vi "rs3_cull_obj2.vi"(7 "file path (dialog if empty)":path=path "C:/ProgramData/Obj_and_PNG_Recording/FacePointCloud_4.obj", 10 "all faces input":i32[][](array[numeric])=array65200x3[195600 elements], 11 "vertices":dbl[][](array[numeric])=array32964x6[197784 elements]) -> (2 "New Faces (proper index)":dbl[][](array[numeric]), 3 "new vertices":dbl[][](array[numeric]))   [LabVIEW 2017, in "libRealSense3.lvlib"]
uses:
  <vilib>/Utility/file.llb/Write Delimited Spreadsheet (string).vi
  libRealSense3.lvlib
panel:
  out "depth array":dbl[](array[numeric])
  out "Good faces":bool[](array[boolean])
  out "Valid vertices":bool[](array[boolean])
  out "New valid faces":i32[][](array[numeric])
  out "Offset":dbl[](array[numeric])
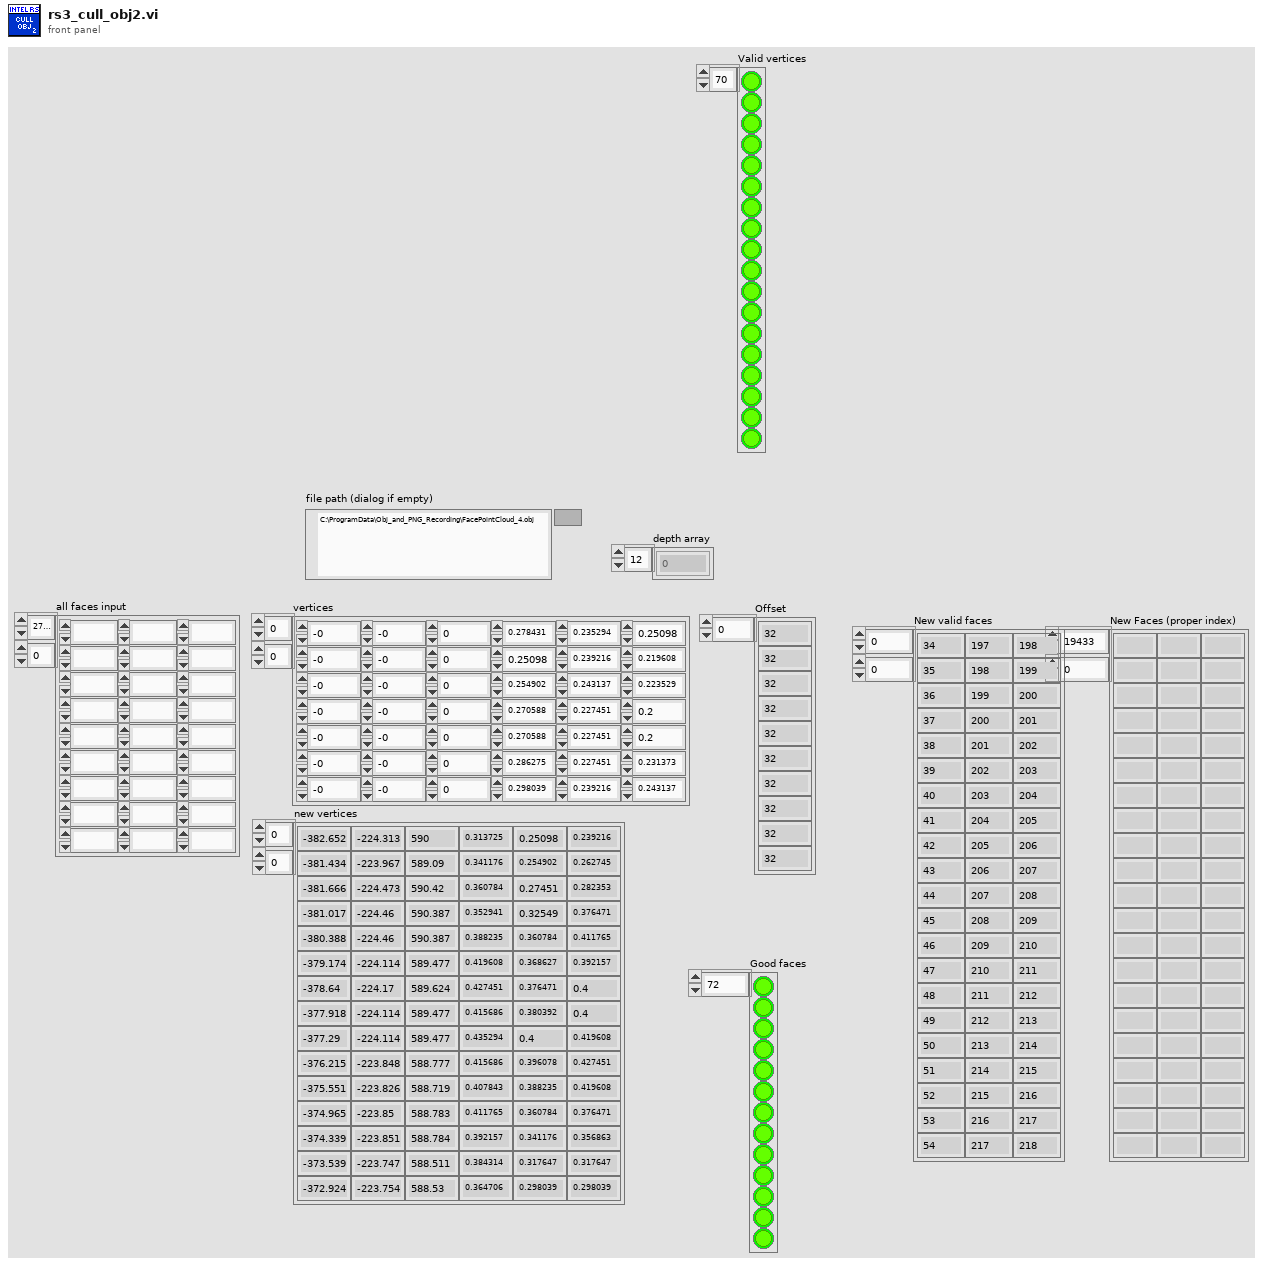
[diagram p1: front panel]
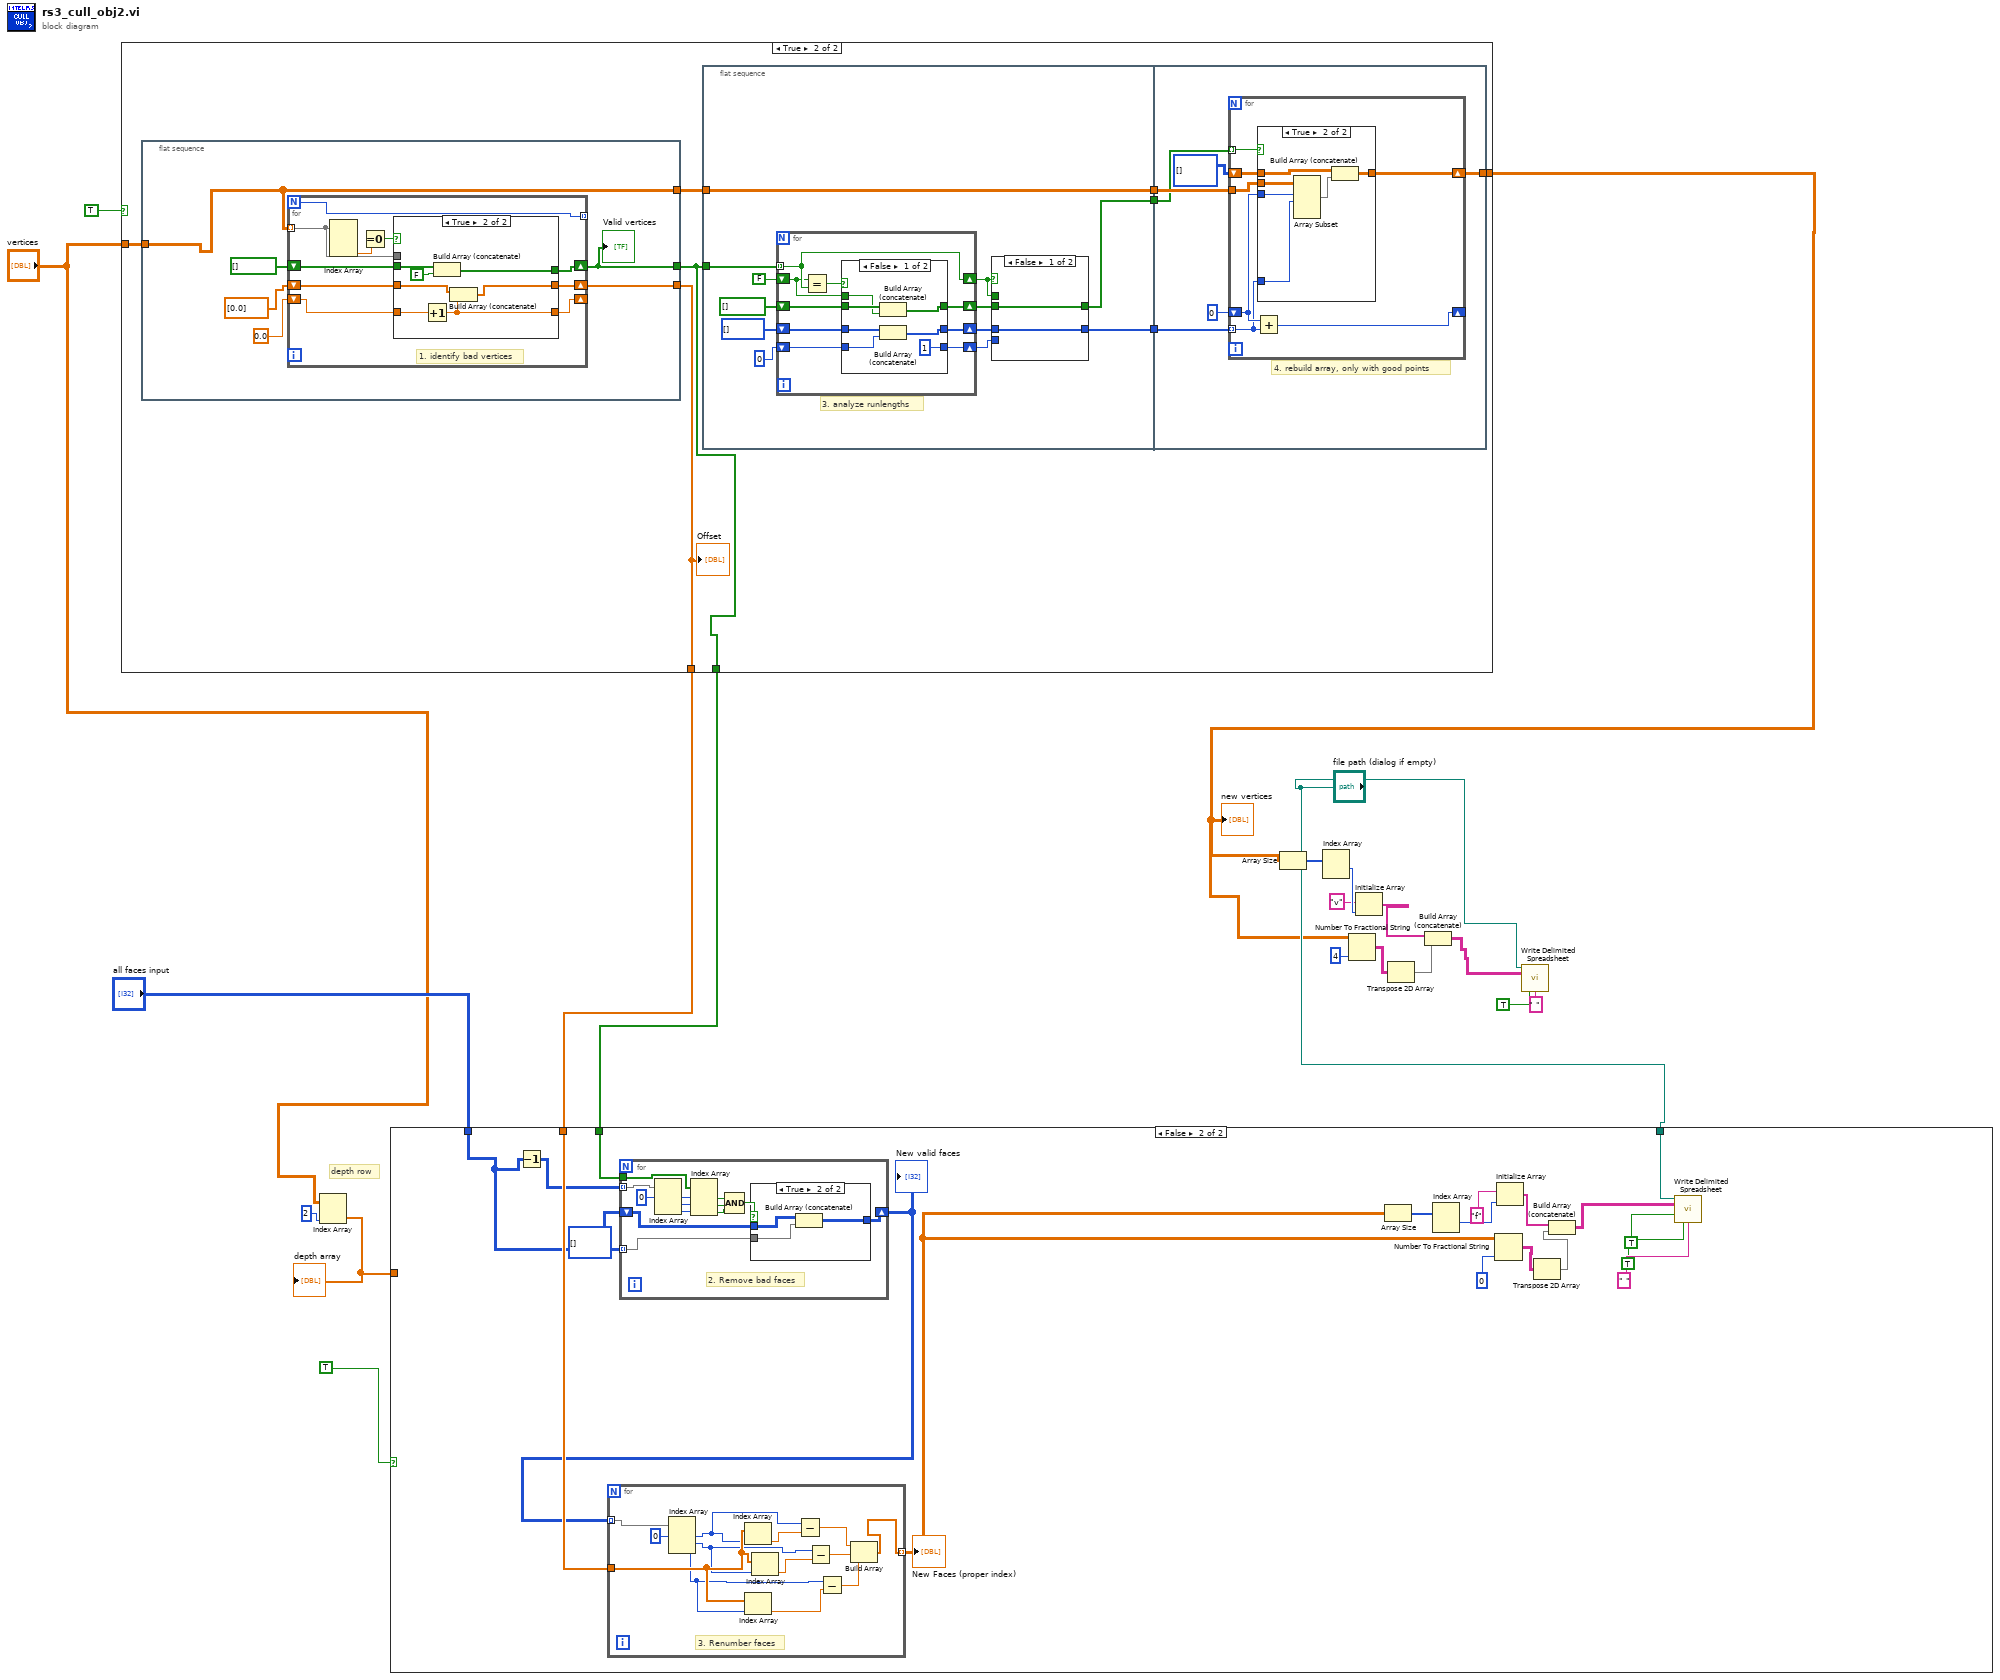
[diagram p0: block diagram]
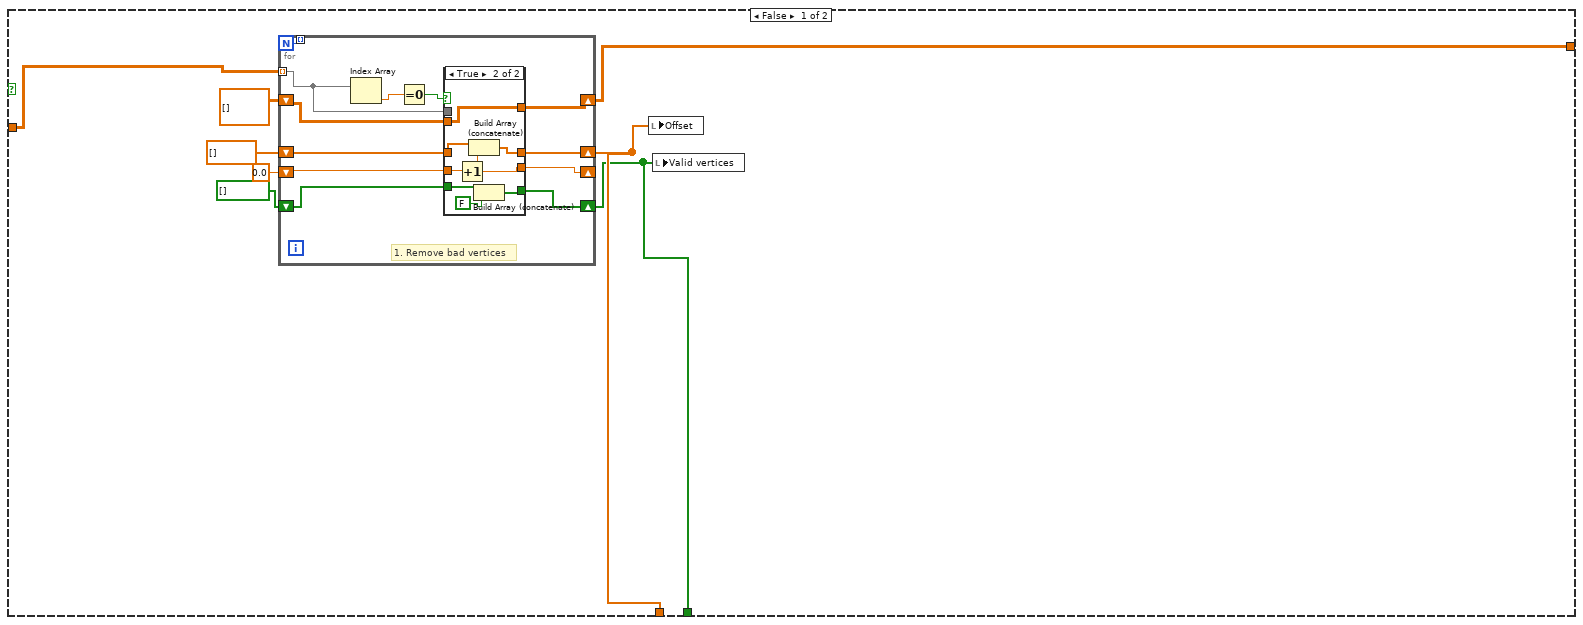
[diagram p2: hidden frame]
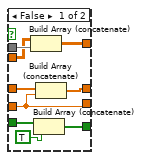
[diagram p3: hidden frame]
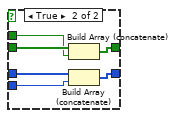
[diagram p4: hidden frame]
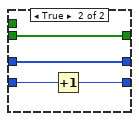
[diagram p5: hidden frame]
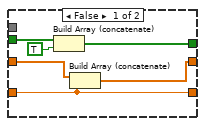
[diagram p7: hidden frame]
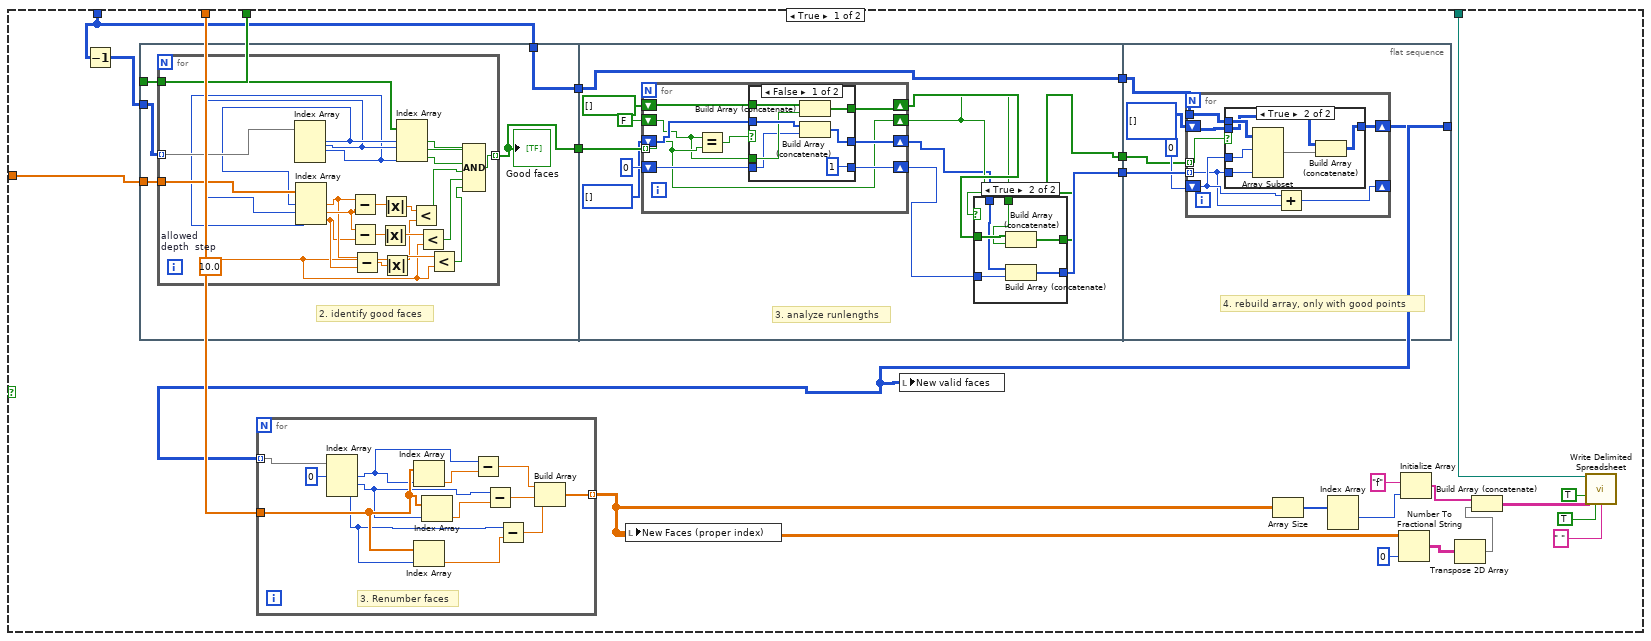
[diagram p8: hidden frame]
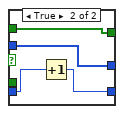
[diagram p10: hidden frame]
diagram:
  # "depth row"
  n1 = case shown="True" TRUE {
    tunnel: [w22 w61] -> w7
    tunnel: "vertices" -> [w24 w60]
    tunnel: [w23 w58] -> w5
    tunnel: [w21 w59] -> w4
    frame False {
      n2 = for {
        N -> [w31]
        tunnel: w24 -> [w40] mode=indexing
        shift-right: [w39] -> w22
        shift-left: dbl[][] [] -> [w37]
        shift-right: [w32] -> w23
        shift-left: dbl[] [] -> [w35]
        shift-right: [w33] -> _
        shift-left: 0.0 -> [w34]
        tunnel: [w31] -> _ mode=indexing
        shift-right: [w29] -> w21
        shift-left: bool[] [] -> [w30]
        # "1. Remove bad vertices"
        n3 = Index Array(array=w40) -> (element=w36:dbl)  [unwired: 1 in]
        n4 = Equal To 0?(x=w36) -> (x = 0?=w38:bool)
        n5 = case shown="True" w38 {
          tunnel: w40 -> [w49 _]
          tunnel: [w48 w57] -> w39
          tunnel: w37 -> [w47 w57]
          tunnel: w35 -> [w46 w52]
          tunnel: w34 -> [w45 w56]
          tunnel: [w45 w51] -> w33
          tunnel: [w44 w50] -> w32
          tunnel: [w43 w53] -> w29
          tunnel: w30 -> [w41 w55]
          frame False {
            n6 = Build Array (concatenate)(w47, w49) -> (w48:dbl[][])
            n7 = Build Array (concatenate)(w41, TRUE) -> (w43:bool[])
            n8 = Build Array (concatenate)(w46, w45) -> (w44:dbl[])
          }
          frame True {
            n9 = Increment(x=w56) -> (x+1=w51:dbl)
            n10 = Build Array (concatenate)(w52, w51) -> (w50:dbl[])
            n11 = Build Array (concatenate)(w55, FALSE) -> (w53:bool[])
          }
        }
      }
      n12 = local write "Offset"(w23) -> ()
      n13 = local write "Valid vertices"(w21) -> ()
    }
    frame True {
      n14 = flat-sequence {
        tunnel: [w130] -> w59
        tunnel: [w129] -> w62
        tunnel: w60 -> [w129]
        tunnel: [w126] -> w58
        frame #0 {
          n15 = for {
            N -> [w139]
            tunnel: w129 -> [w141] mode=indexing
            tunnel: [w139] -> _ mode=indexing
            shift-right: [w137] -> w130
            shift-left: bool[] [] -> [w138]
            shift-right: [w133] -> w126
            shift-left: dbl[] [0.0] -> [w135]
            shift-right: [w132] -> _
            shift-left: 0.0 -> [w134]
            # "1. identify bad vertices"
            n16 = Index Array(array=w141) -> (element #3=w136:dbl)  [unwired: 3 in, 2 out]
            n17 = Equal To 0?(x=w136) -> (x = 0?=w140:bool)
            n18 = case shown="True" w140 {
              tunnel: w141 -> [_ _]
              tunnel: [w147 w152] -> w137
              tunnel: w138 -> [w145 w154]
              tunnel: w135 -> [w144 w151]
              tunnel: w134 -> [w142 w149]
              tunnel: [w143 w150] -> w133
              tunnel: [w142 w148] -> w132
              frame False {
                n19 = Build Array (concatenate)(w145, TRUE) -> (w147:bool[])
                n20 = Build Array (concatenate)(w144, w142) -> (w143:dbl[])
              }
              frame True {
                n21 = Increment(x=w149) -> (x+1=w148:dbl)
                n22 = Build Array (concatenate)(w154, FALSE) -> (w152:bool[])
                n23 = Build Array (concatenate)(w151, w148) -> (w150:dbl[])
              }
            }
          }
          "Valid vertices" <- w130
        }
      }
      n24 = flat-sequence {
        tunnel: [w67] -> w65
        tunnel: [w68] -> w64
        tunnel: [w69] -> w63
        tunnel: w62 -> [w67]
        tunnel: w59 -> [w66]
        tunnel: w65 -> [w111]
        tunnel: w64 -> [w108]
        tunnel: w63 -> [w110]
        tunnel: [w106] -> w61
        frame #0 {
          # "3. analyze runlengths"
          n25 = for {
            tunnel: w66 -> [w89] mode=indexing
            shift-right: [w89] -> w72
            shift-left: FALSE -> [w86]
            shift-right: [w93] -> w70
            shift-left: 0 -> [w94]
            shift-right: [w92] -> w71
            shift-left: i32[] [] -> [w91]
            shift-right: [w87] -> w73
            shift-left: bool[] [] -> [w88]
            n26 = Equal?(x=w86, y=w89) -> (x = y?=w90:bool)
            n27 = case shown="False" w90 {
              tunnel: w94 -> [w95 w105]
              tunnel: [1 w104] -> w93
              tunnel: [w100 w103] -> w92
              tunnel: w91 -> [w99 w103]
              tunnel: w88 -> [w98 w102]
              tunnel: [w97 w102] -> w87
              tunnel: w86 -> [w96 _]
              frame False {
                n28 = Build Array (concatenate)(w98, w96) -> (w97:bool[])
                n29 = Build Array (concatenate)(w99, w95) -> (w100:i32[])
              }
              frame True {
                n30 = Increment(x=w105) -> (x+1=w104:i32)
              }
            }
          }
          n31 = case shown="False" w72 {
            tunnel: w73 -> [w79 w85]
            tunnel: w72 -> [_ w84]
            tunnel: w71 -> [w78 w83]
            tunnel: w70 -> [_ w82]
            tunnel: [w78 w81] -> w69
            tunnel: [w79 w80] -> w68
            frame False {
            }
            frame True {
              n32 = Build Array (concatenate)(w85, w84) -> (w80:bool[])
              n33 = Build Array (concatenate)(w83, w82) -> (w81:i32[])
            }
          }
        }
        frame #1 {
          # "4. rebuild array, only with good points"
          n34 = for {
            shift-right: [w116] -> _
            shift-left: 0 -> [w117]
            tunnel: w111 -> [w118]
            tunnel: w110 -> [w115] mode=indexing
            shift-right: [w112] -> w106
            shift-left: i32[][] [] ("all faces input") -> [w114]
            tunnel: w108 -> [w113] mode=indexing
            n35 = Add(x=w117, y=w115) -> (x+y=w116:i32)
            n36 = case shown="True" w113 {
              tunnel: w118 -> [_ w125]
              tunnel: w117 -> [_ w124]
              tunnel: w115 -> [_ w122]
              tunnel: w114 -> [w119 w120]
              tunnel: [w119 w121] -> w112
              frame False {
              }
              frame True {
                n37 = Array Subset(array=w125, index (row)=w124, length (row)=w122) -> (w123:dbl[][])  [unwired: 2 in]
                n38 = Build Array (concatenate)(w120, w123) -> (w121:dbl[][])
              }
            }
          }
        }
      }
      "Offset" <- w58
    }
  }
  "new vertices" <- w7
  n39 = Index Array(array="vertices", index (col)=2 ("index (row)")) -> (element=w2:dbl[])  [unwired: 1 in]
  "depth array" <- w2
  n40 = case shown="False" TRUE {
    tunnel: w4 -> [w160 w297]
    tunnel: "file path (dialog if empty)" -> [w169 w287]
    tunnel: w5 -> [w166 w284]
    tunnel: "all faces input" -> [w158 w281]
    tunnel: w2 -> [w155 _]
    frame True {
      n41 = Decrement(x=w158) -> (x-1=w159:i32[][])
      n42 = flat-sequence {
        tunnel: w160 -> [w183]
        tunnel: w159 -> [w182]
        tunnel: [w181] -> w165
        tunnel: w158 -> [w181]
        tunnel: [w180] -> w164
        tunnel: w155 -> [w179]
        tunnel: w165 -> [w215]
        tunnel: w164 -> [w218]
        tunnel: [w215] -> w163
        tunnel: [w207] -> w162
        tunnel: [w208] -> w161
        tunnel: w163 -> [w252]
        tunnel: w162 -> [w249]
        tunnel: w161 -> [w251]
        tunnel: [w247] -> w157
        frame #0 {
          # "2. identify good faces"
          n43 = for {
            tunnel: w182 -> [w206] mode=indexing
            tunnel: w183 -> [w205]
            tunnel: [w201] -> w180 mode=indexing
            tunnel: w179 -> [w200]
            w192 = 10.0  # allowed  depth  step
            n44 = Index Array(array=w206) -> (element #1=w186:i32, element #2=w184:i32, element #3=w185:i32)  [unwired: 3 in]
            n45 = Index Array(array=w200, index #1=w186, index #2=w185, index #3=w184) -> (element #1=w198:dbl, element #2=w199:dbl, element #3=w197:dbl)
            n46 = Subtract(x=w198, y=w199) -> (x-y=w191:dbl)
            n47 = Subtract(x=w199, y=w197) -> (x-y=w196:dbl)
            n48 = Subtract(x=w198, y=w197) -> (x-y=w195:dbl)
            n49 = Absolute Value(x=w196) -> (abs(x)=w194:dbl)
            n50 = Absolute Value(x=w191) -> (abs(x)=w190:dbl)
            n51 = Absolute Value(x=w195) -> (abs(x)=w193:dbl)
            n52 = Index Array(array=w205, index #1=w186, index #2=w184, index #3=w185) -> (element #1=w204:bool, element #2=w203:bool, element #3=w202:bool)
            n53 = Less?(x=w190, y=w192) -> (x < y?=w189:bool)
            n54 = Less?(x=w194, y=w192) -> (x < y?=w188:bool)
            n55 = Less?(x=w193, y=w192) -> (x < y?=w187:bool)
            n56 = Compound Arithmetic op=AND(w204, w203, w202, w189, w188, w187) -> (w201:bool)
          }
          "Good faces" <- w180
        }
        frame #1 {
          # "3. analyze runlengths"
          n57 = for {
            tunnel: w218 -> [w230] mode=indexing
            shift-right: [w230] -> w211
            shift-left: FALSE -> [w227]
            shift-right: [w234] -> w209
            shift-left: 0 -> [w235]
            shift-right: [w233] -> w210
            shift-left: i32[] [] -> [w232]
            shift-right: [w228] -> w212
            shift-left: bool[] [] -> [w229]
            n58 = Equal?(x=w227, y=w230) -> (x = y?=w231:bool)
            n59 = case shown="False" w231 {
              tunnel: w235 -> [w236 w246]
              tunnel: [1 w245] -> w234
              tunnel: [w241 w244] -> w233
              tunnel: w232 -> [w240 w244]
              tunnel: w229 -> [w239 w243]
              tunnel: [w238 w243] -> w228
              tunnel: w227 -> [w237 _]
              frame False {
                n60 = Build Array (concatenate)(w239, w237) -> (w238:bool[])
                n61 = Build Array (concatenate)(w240, w236) -> (w241:i32[])
              }
              frame True {
                n62 = Increment(x=w246) -> (x+1=w245:i32)
              }
            }
          }
          n63 = case shown="True" w211 {
            tunnel: w212 -> [w220 w226]
            tunnel: w211 -> [_ w225]
            tunnel: w210 -> [w219 w224]
            tunnel: w209 -> [_ w223]
            tunnel: [w219 w222] -> w208
            tunnel: [w220 w221] -> w207
            frame False {
            }
            frame True {
              n64 = Build Array (concatenate)(w226, w225) -> (w221:bool[])
              n65 = Build Array (concatenate)(w224, w223) -> (w222:i32[])
            }
          }
        }
        frame #2 {
          # "4. rebuild array, only with good points"
          n66 = for {
            shift-right: [w257] -> _
            shift-left: 0 -> [w258]
            tunnel: w252 -> [w259]
            tunnel: w251 -> [w256] mode=indexing
            shift-right: [w253] -> w247
            shift-left: i32[][] [] ("all faces input") -> [w255]
            tunnel: w249 -> [w254] mode=indexing
            n67 = case shown="True" w254 {
              tunnel: w259 -> [_ w266]
              tunnel: w258 -> [_ w265]
              tunnel: w256 -> [_ w263]
              tunnel: w255 -> [w260 w261]
              tunnel: [w260 w262] -> w253
              frame False {
              }
              frame True {
                n68 = Array Subset(array=w266, index (row)=w265, length (row)=w263) -> (w264:i32[][])  [unwired: 2 in]
                n69 = Build Array (concatenate)(w261, w264) -> (w262:i32[][])
              }
            }
            n70 = Add(x=w258, y=w256) -> (x+y=w257:i32)
          }
        }
      }
      n71 = for {
        tunnel: w157 -> [w279] mode=indexing
        tunnel: w166 -> [w273]
        tunnel: [w275] -> w156 mode=indexing
        # "3. Renumber faces"
        n72 = Index Array(array=w279, index #1=0 ("index")) -> (element #1=w267:i32, element #2=w270:i32, element #3=w272:i32)  [unwired: 2 in]
        n73 = Index Array(array=w273, index=w267) -> (element=w268:dbl)
        n74 = Index Array(array=w273, index=w272) -> (element=w271:dbl)
        n75 = Index Array(array=w273, index=w270) -> (element=w274:dbl)
        n76 = Subtract(x=w267, y=w268) -> (x-y=w278:dbl)
        n77 = Subtract(x=w270, y=w274) -> (x-y=w277:dbl)
        n78 = Subtract(x=w272, y=w271) -> (x-y=w276:dbl)
        n79 = Build Array(w278, w277, w276) -> (w275:dbl[])
      }
      n80 = local write "New Faces (proper index)"(w156) -> ()
      n81 = local write "New valid faces"(w157) -> ()
      n82 = Array Size(array=w156) -> (size(s)=w178:i32[])
      n83 = Index Array(array=w178) -> (element #1=w176:i32)  [unwired: 2 in, 1 out]
      n84 = Number To Fractional String(number=w156, precision (6)=i16 0) -> (F-format string=w173:string[][])  [unwired: 2 in]
      n85 = Initialize Array("f", w176) -> (w174:string[])
      n86 = Transpose 2D Array(2D array=w173) -> (transposed array=w172:string[][])
      n87 = Build Array (concatenate)(w174, w172) -> (w167:string[][])
      n88 = call-poly <vilib>:"Write Delimited Spreadsheet.vi"("file path (dialog if empty)"=w169, "2D data"=w167, "append to file? (new file:F)"=TRUE ("append to file? (F)"), "transpose? (no:F)"=TRUE ("transpose? (F)"), "delimiter (\\t)"=" " ("delimiter (\\t)")) -> ()  [unwired: 9 in, 2 out]
    }
    frame False {
      n89 = Decrement(x=w281) -> (x-1=w280:i32[][])
      n90 = for {
        tunnel: w281 -> [w311] mode=indexing
        shift-right: [w310] -> w283
        shift-left: i32[][] [] -> [w309]
        tunnel: w297 -> [w308]
        tunnel: w280 -> [w299] mode=indexing
        # "2. Remove bad faces"
        n91 = Index Array(array=w299, index #1=0 ("index")) -> (element #1=w307:i32, element #2=w306:i32, element #3=w305:i32)  [unwired: 2 in]
        n92 = Index Array(array=w308, index #1=w307, index #2=w306, index #3=w305) -> (element #1=w304:bool, element #2=w303:bool, element #3=w302:bool)
        n93 = Compound Arithmetic op=AND(w304, w303, w302) -> (w301:bool)
        n94 = case shown="True" w301 {
          tunnel: w311 -> [_ w315]
          tunnel: [w312 w314] -> w310
          tunnel: w309 -> [w312 w313]
          frame False {
          }
          frame True {
            n95 = Build Array (concatenate)(w313, w315) -> (w314:i32[][])
          }
        }
      }
      "New valid faces" <- w283
      n96 = for {
        tunnel: w283 -> [w328] mode=indexing
        tunnel: w284 -> [w323]
        tunnel: [w316] -> w282 mode=indexing
        # "3. Renumber faces"
        n97 = Index Array(array=w328, index #1=0 ("index")) -> (element #1=w317:i32, element #2=w320:i32, element #3=w322:i32)  [unwired: 2 in]
        n98 = Index Array(array=w323, index=w317) -> (element=w318:dbl)
        n99 = Index Array(array=w323, index=w322) -> (element=w321:dbl)
        n100 = Index Array(array=w323, index=w320) -> (element=w324:dbl)
        n101 = Subtract(x=w317, y=w318) -> (x-y=w327:dbl)
        n102 = Subtract(x=w320, y=w324) -> (x-y=w326:dbl)
        n103 = Subtract(x=w322, y=w321) -> (x-y=w325:dbl)
        n104 = Build Array(w327, w326, w325) -> (w316:dbl[])
      }
      "New Faces (proper index)" <- w282
      n105 = Array Size(array=w282) -> (size(s)=w296:i32[])
      n106 = Index Array(array=w296) -> (element #1=w294:i32)  [unwired: 2 in, 1 out]
      n107 = Number To Fractional String(number=w282, precision (6)=i16 0) -> (F-format string=w291:string[][])  [unwired: 2 in]
      n108 = Initialize Array("f", w294) -> (w292:string[])
      n109 = Transpose 2D Array(2D array=w291) -> (transposed array=w290:string[][])
      n110 = Build Array (concatenate)(w292, w290) -> (w285:string[][])
      n111 = call-poly <vilib>:"Write Delimited Spreadsheet.vi"("file path (dialog if empty)"=w287, "2D data"=w285, "append to file? (new file:F)"=TRUE ("append to file? (F)"), "transpose? (no:F)"=TRUE ("transpose? (F)"), "delimiter (\\t)"=" " ("delimiter (\\t)")) -> ()  [unwired: 9 in, 2 out]
    }
  }
  n112 = Array Size(array=w7) -> (size(s)=w17:i32[])
  n113 = Index Array(array=w17) -> (element #1=w16:i32)  [unwired: 2 in, 1 out]
  n114 = Number To Fractional String(number=w7, precision (6)=i16 4) -> (F-format string=w10:string[][])  [unwired: 2 in]
  n115 = Initialize Array("v", w16) -> (w11:string[])
  n116 = Transpose 2D Array(2D array=w10) -> (transposed array=w9:string[][])
  n117 = Build Array (concatenate)(w11, w9) -> (w8:string[][])
  n118 = call-poly <vilib>:"Write Delimited Spreadsheet.vi"("file path (dialog if empty)"="file path (dialog if empty)", "2D data"=w8, "transpose? (no:F)"=TRUE ("transpose? (F)"), "delimiter (\\t)"=" " ("delimiter (\\t)")) -> ()  [unwired: 10 in, 2 out]
